vi "UHR-Fleezers Control (host) - 12.8.1.vi"() -> ()   [LabVIEW 2012] (continued)
                  frame Disabled {
                  }
                  frame Enabled {
                  }
                }
                n1750 = local read "Actual MCL Inc (V)"() -> (w2644:dbl)
                n1751 = local read "Scan steps (MCL)"() -> (w2649:u64)
                n1752 = Divide "Y Pix/step"(x=w2645, y=w2650) -> (x/y=w2657:dbl)
                n1753 = Divide "Y V/pix"(x=w2644, y=w2657) -> (x/y=w2656:dbl)
                n1754 = Divide "Y half step offset"(x=w2644, y=2.0) -> (x/y=w2658:dbl)
                n1755 = Divide "X pix/step"(x=w2646, y=w2649) -> (x/y=w2655:dbl)
                n1756 = Negate(x=w2658) -> (-x=w2659:dbl)
                n1757 = local read "Initial Y"() -> (w2665:dbl)
                n1758 = Multiply(x=w2647, y=w2656) -> (x*y=w2666:dbl)
                n1759 = Divide "X half step offset"(x=w2644, y=2.0) -> (x/y=w2652:dbl)
                n1760 = Divide "X V/pix"(x=w2644, y=w2655) -> (x/y=w2654:dbl)
                n1761 = Multiply(x=w2644, y=w2649) -> (x*y=w2661:dbl)
                n1762 = Compound Arithmetic op=ADD(w2659, w2666, w2665) -> (w2636:dbl)
                "Pointer Y (V)" <- w2636
                n1763 = Multiply(x=w2654, y=w2648) -> (x*y=w2663:dbl)
                n1764 = Negate(x=w2652) -> (-x=w2651:dbl)
                n1765 = local read "Initial X"() -> (w2664:dbl)
                n1766 = Negate(x=w2663) -> (-x=w2662:dbl)
                n1767 = Compound Arithmetic op=ADD(w2651, w2661, w2664, w2662) -> (w2637:dbl)
                "Pointer X (V)" <- w2637
                n1768 = case shown="True" "Set High F Confocal Spot (X-Y)" {
                  tunnel: w2637 -> [_ w2667]
                  tunnel: w2636 -> [_ w2668]
                  frame False {
                  }
                  frame True {
                    "Confocal Y 2 (V)" <- w2668
                    "Confocal X 2 (V)" <- w2667
                  }
                }
                n1769 = Or(x="Set X Only", y="Set Confocal Spot (X-Y)") -> (x .or. y?=w2640:bool)
                n1770 = Or(x="Set Confocal Spot (X-Y)", y="Set Y Only") -> (x .or. y?=w2639:bool)
                n1771 = case shown="True" w2640 {
                  tunnel: w2637 -> [_ w2669]
                  frame False {
                  }
                  frame True {
                    n1772 = property on="AO2" class="Slide (strict)"("Val(Sgnl)"=w2669) -> ()  [unwired: 2 in, 2 out]
                    "Confocal X 1 (V)" <- w2669
                  }
                }
                n1773 = case shown="True" w2639 {
                  tunnel: w2636 -> [_ w2670]
                  frame False {
                  }
                  frame True {
                    n1774 = property on="AO1" class="Slide (strict)"("Val(Sgnl)"=w2670) -> ()  [unwired: 2 in, 2 out]
                    "Confocal Y 1 (V)" <- w2670
                  }
                }
                n1775 = local write "Set High F Confocal Spot (X-Y)"(w2635) -> ()
                n1776 = local write "Set Confocal Spot (X-Y)"(w2635) -> ()
                n1777 = local write "Set X Only"(w2635) -> ()
                n1778 = local write "Set Y Only"(w2635) -> ()
              }
            }
          }
          frame 3 {
            n1779 = local read "BD 2 Frequency 1 (MHz)"() -> (w2672:dbl)
            n1780 = local read "BD 1 Frequency 1 (MHz)"() -> (w2673:dbl)
            n1781 = local write "Manipulating Trap"(TRUE ("Manipulating Trap")) -> ()
            n1782 = local write "Coords"(T9 {"Horizontal"=0, "Vertical"=0} ("Coords")) -> ()
            n1783 = while {
              tunnel: w2677 -> [w2682]
              tunnel: w2675 -> [w2681]
              tunnel: w2673 -> [w2680]
              tunnel: w2672 -> [w2679]
              tunnel: w2671 -> [w2678]
              stop <- w2683 stop-if-true
              n1784 = event shown="[0] \"Pane\": Mouse Move" {
                selector: _ -> [_ _]
                dyn-events: _ -> [_ _]
                timeout: _ -> [_ _]
                tunnel: ["Force Manip Abort" w2747] -> w2683
                tunnel: w2682 -> [w2690 _]
                tunnel: w2681 -> [w2688 _]
                tunnel: w2680 -> [w2687 _]
                tunnel: w2679 -> [w2686 _]
                tunnel: w2678 -> [w2684 _]
                event Mouse Move {
                  n1785 = event-data() -> ("Time"=w2691:u32, "Coords"=w2692:T9)  [unwired: 3 out]
                  n1786 = Less?(x=w2691, y=w2690) -> (x < y?=w2689:bool)
                  n1787 = case "Makes sure old motion events prior to mouse click aren't used" shown="False" w2689 {
                    tunnel: w2692 -> [w2734 _]
                    tunnel: w2688 -> [w2735 _]
                    tunnel: w2687 -> [w2709 _]
                    tunnel: w2686 -> [w2708 _]
                    tunnel: w2684 -> [w2693 _]
                    frame False {
                      n1788 = Subtract(x=w2734, y=w2735) -> (x-y=w2733:T9)
                      "Coords" <- w2733
                      n1789 = local read "Y RF Frequency Limits (MHz)"() -> (w2694:T18)
                      n1790 = To Double Precision Float(number=w2733) -> (double precision float=w2732:cluster{"Horizontal":dbl, "Vertical":dbl})
                      n1791 = Multiply(x=cluster{"Horizontal":dbl, "Vertical":dbl} {"Horizontal"=-1.0, "Vertical"=1.0}, y="Manipulation Scaling") -> (x*y=w2728:cluster{"Horizontal":dbl, "Vertical":dbl})
                      n1792 = local read "X RF Frequency Limits (MHz)"() -> (w2695:T18)
                      n1793 = Multiply(x=w2732, y=w2728) -> (x*y=w2730:cluster{"Horizontal":dbl, "Vertical":dbl})
                      n1794 = Unbundle By Name(w2730) -> ("Horizontal"=w2725:dbl, "Vertical"=w2729:dbl)
                      n1795 = Unbundle By Name(w2694) -> ("Maximum"=w2697:dbl, "Minimum"=w2696:dbl)
                      n1796 = Boolean To (0,1)(Boolean="Manip. X?") -> (0, 1=w2723:i16)
                      n1797 = Boolean To (0,1)(Boolean="Manip. Y?") -> (0, 1=w2720:i16)
                      n1798 = local read "BD 1 Frequency 2 (MHz)"() -> (w2711:dbl)
                      n1799 = Multiply(x=w2729, y=w2720) -> (x*y=w2722:dbl)
                      n1800 = Multiply(x=w2723, y=w2725) -> (x*y=w2726:dbl)
                      n1801 = local read "BD 2 Frequency 2 (MHz)"() -> (w2710:dbl)
                      n1802 = Unbundle By Name(w2695) -> ("Maximum"=w2699:dbl, "Minimum"=w2698:dbl)
                      n1803 = Add(x=w2708, y=w2722) -> (x+y=w2701:dbl)
                      n1804 = Add(x=w2709, y=w2726) -> (x+y=w2703:dbl)
                      n1805 = In Range and Coerce(upper limit=w2699, x=w2703, lower limit=w2698) -> (coerced(x)=w2702:dbl)  [unwired: 1 out]
                      n1806 = In Range and Coerce(upper limit=w2697, x=w2701, lower limit=w2696) -> (coerced(x)=w2700:dbl)  [unwired: 1 out]
                      n1807 = Subtract(x=w2702, y=w2711) -> (x-y=w2719:dbl)
                      n1808 = Subtract(x=w2700, y=w2710) -> (x-y=w2718:dbl)
                      n1809 = Square(x=w2719) -> (x^2=w2717:dbl)
                      n1810 = Square(x=w2718) -> (x^2=w2716:dbl)
                      n1811 = Add(x=w2717, y=w2716) -> (x+y=w2715:dbl)
                      n1812 = Square Root(x=w2715) -> (sqrt(x)=w2712:dbl)
                      n1813 = In Range and Coerce(upper limit="Limit Max (MHz)", x=w2712, lower limit="Limit Min (MHz)") -> (In Range?=w2705:bool)  [unwired: 1 out]
                      n1814 = Not(x="Limits Enable") -> (.not. x?=w2704:bool)
                      n1815 = Or(x=w2705, y=w2704) -> (x .or. y?=w2706:bool)
                      n1816 = case shown="True" w2706 {
                        tunnel: w2712 -> [_ w2737]
                        tunnel: w2702 -> [_ w2744]
                        tunnel: w2711 -> [_ w2743]
                        tunnel: w2700 -> [_ w2742]
                        tunnel: w2710 -> [_ w2741]
                        tunnel: w2695 -> [_ w2739]
                        tunnel: w2694 -> [_ w2738]
                        tunnel: w2693 -> [_ w2736]
                        frame False {
                        }
                        frame True {
                          n1817 = local read "BD 1 Frequency 3 (MHz)"() -> (w2745:dbl)
                          n1818 = local read "BD 2 Frequency 3 (MHz)"() -> (w2740:dbl)
                          n1819 = local write "Trap Delta (MHz)"(w2737) -> ()
                          n1820 = call "set RF board frequency - interlace.vi"("Board 2 Frequency Limits"=w2738, "Board 1 Frequency Limits"=w2739, "FPGA VI Reference In"=w2736, "Board 2 Frequency 3 (MHz)"=w2740, "Board 1 Frequency 3 (MHz)"=w2745, "Board 2 Frequency 2 (MHz)"=w2741, "Board 2 Frequency 1 (MHz)"=w2742, "Board 1 Frequency 2 (MHz)"=w2743, "Board 1 Frequency 1  (MHz)"=w2744) -> ()  [unwired: 1 in, 2 out]
                          n1821 = local write "BD 2 Frequency 1 (MHz)"(w2742) -> ()
                          n1822 = local write "BD 1 Frequency 1 (MHz)"(w2744) -> ()
                        }
                      }
                    }
                    frame True {
                    }
                  }
                }
                event Mouse Up {
                  n1823 = event-data() -> ("Button"=w2746:u16)  [unwired: 8 out]
                  n1824 = case shown="3" w2746 {
                    tunnel: [FALSE TRUE] -> w2747
                    frame 0, Default {
                    }
                    frame 3 {
                      n1825 = local read "Trap Delta (MHz)"() -> (w2749:dbl)
                      n1826 = property on="Initial delta (MHz)" class="DigNum (strict)"("Val(Sgnl)"=w2749) -> ()  [unwired: 2 in, 2 out]
                      n1827 = local write "Manipulating Trap"(FALSE ("Manipulating Trap")) -> ()
                    }
                  }
                }
              }
            }
          }
        }
      }
      event Mouse Move {
        n1828 = event-data() -> ()  [unwired: 6 out]
      }
    }
    n1829 = local read "Stop All"() -> (w2565:bool)
    n1830 = node-c288() -> ()  [unwired: 2 out]
  }
  n1831 = flat-sequence "Video" {
    tunnel: [w2762] -> w67
    tunnel: w67 -> [w2803]
    frame #0 {
      w2752 = FALSE ("File open?")
      n1832 = while {
        stop <- w2754 continue-if-true
        n1833 = call "Close Video Capture.vi"() -> ("error code OUT"=w2756:i32)
        n1834 = Equal?(x=w2756, y=0) -> (x = y?=w2754:bool)
      }
      n1835 = local write "New Video File"(w2752) -> ()
      n1836 = local write "File open?"(w2752) -> ()
      n1837 = local write "Save Video"(w2752) -> ()
      n1838 = local write "Stop All"(FALSE ("Stop All")) -> ()
    }
    frame #1 {
      n1839 = call "DMR_Init.vi"() -> ()  [unwired: 3 out]
    }
    frame #2 {
      w2757 = "DE245428202"  # MSU fleezers card #
      (unwired) "DE019116701"  # Illinois fleezers card #
      # "Setting the destination format to Mono8 makes sure that the image can be displayed in the intensity plot."
      n1840 = call "DMR_GetDevice.vi"("search string IN"=w2757) -> ("device handle OUT"=w2780:i32)  [unwired: 4 in, 2 out]
      n1841 = call "DMR_OpenDevice.vi"("device handle IN"=w2780) -> ("driver handle OUT"=w2763:i32)  [unwired: 4 out]
      n1842 = call "DMR_FindList.vi"("flags IN"=u32 0 ("flags"), "list name IN"="" ("String"), "list type IN"=T39."camera descriptions", "driver handle IN"=w2763) -> ("list handle OUT"=w2766:i32)  [unwired: 2 out]
      n1843 = call "DMR_FindList.vi"("flags IN"=u32 0 ("flags"), "list name IN"="Base", "list type IN"=T39."setting", "driver handle IN"=w2763) -> ("list handle OUT"=w2764:i32)  [unwired: 2 out]
      n1844 = call "OBJ_GetHandle.vi"("object name IN"="VideoStandard", "list handle IN"=w2766) -> ("object handle OUT"=w2760:i32)  [unwired: 3 out]
      n1845 = call "OBJ_GetHandle.vi"("object name IN"="PixelFormat", "list handle IN"=w2764) -> ("object handle OUT"=w2774:i32)  [unwired: 3 out]
      n1846 = call "OBJ_SetS.vi"("value index IN"=0, "value IN"="NTSC M", "object handle IN"=w2760) -> ()  [unwired: 2 out]
      n1847 = call "OBJ_SetS.vi"("value index IN"=0, "value IN"="Mono8" ("value"), "object handle IN"=w2774) -> ()  [unwired: 2 out]
      n1848 = call "OBJ_GetHandle.vi"("object name IN"="VideoChannel", "list handle IN"=w2764) -> ("object handle OUT"=w2770:i32)  [unwired: 3 out]
      n1849 = while {
        tunnel: [w2784] -> w2762
        tunnel: w2763 -> [w2781]
        stop <- w2782 continue-if-true
        n1850 = call "DMR_ImageRequestSingle.vi"("request control IN"=0, "driver handle IN"=w2781) -> ("error code OUT"=w2783:i32, "driver handle OUT"=w2784:i32)  [unwired: 2 out]
        n1851 = Equal To 0?(x=w2783) -> (x = 0?=w2782:bool)
      }
      n1852 = call "OBJ_SetI.vi"("value index IN"=0, "value IN"=3 ("Video channel"), "object handle IN"=w2770) -> ()  [unwired: 2 out]
    }
    frame #3 {
      w2791 = T23 0 items=["Grayscale (U8)", "Grayscale (I16)", "Grayscale (SGL)", "Complex (CSG)", "RGB (U32)", "HSL (U32)", "RGB (U64)"] ("Image Type")
      w2799 = T23 0 items=["Grayscale (U8)", "Grayscale (I16)", "Grayscale (SGL)", "Complex (CSG)", "RGB (U32)", "HSL (U32)", "RGB (U64)"] ("Image Type")
      n1853 = call "IMAQ AVI2 Get Codec Names"() -> ("Codec Names"=w2786:string[])  [unwired: 10 in, 1 out]
      "Installed Codec Names" <- w2786
      n1854 = for "Create Greyscale map" {
        N: 256 -> [_]
        tunnel: [w2805] -> w2788 mode=indexing
        workers-P: _ -> [_]
        i -> [w2808]
        n1855 = To Unsigned Byte Integer(number=w2808) -> (unsigned 8bit integer=w2804:u8)
        n1856 = Join Numbers(hi=w2804, lo=w2804) -> ((hi.lo)=w2807:u16)
        n1857 = Join Numbers(hi=w2804, lo=w2804) -> ((hi.lo)=w2806:u16)
        n1858 = Join Numbers(hi=w2807, lo=w2806) -> ((hi.lo)=w2805:u32)
      }
      n1859 = property on="Codec choice" class="CmbBox"("Strings[]"=w2786) -> ()  [unwired: 2 in, 2 out]
      n1860 = call "IMAQ Create"("Image Name"="Scaled video", "Image Type"=w2791) -> ("New Image"=w2790:T2)  [unwired: 2 in, 2 out]
      n1861 = call "IMAQ Create"("Image Name"="Main video", "Image Type"=w2799) -> ("New Image"=w2800:T2)  [unwired: 2 in, 2 out]
      n1862 = node-c288(0 ("Processor")) -> (w2798:T27)  [unwired: 3 out]
      n1863 = Initialize Array(u32 0 ("Window Number (0...15)"), 480 ("dimension size"), 640 ("dimension size")) -> (w2793:u32[][])
      n1864 = timed-loop {
        tunnel: w2803 -> [w2825]
        tunnel: [w2824] -> w2802
        tunnel: w2800 -> [w2823]
        timing: w2798 -> [_]
        timing-out: [_] -> w2797
        tunnel: w2793 -> [w2816]
        tunnel: w2790 -> [w2814]
        tunnel: w2788 -> [w2813]
        stop <- w2815 stop-if-true
        # "This block performs the \nactual image capture."
        n1865 = node-c288() -> (→"Finished Late? [i-1]":bool)  [unwired: 5 out]
        n1866 = local read "Stop All"() -> (w2815:bool)
        n1867 = feedback #1(T40 refnum ("AVI Refnum")) -> (w2821:T40)
        n1868 = case shown="True" "New Video File" {
          tunnel: [w2838 w2839] -> w2812
          tunnel: w2821 -> [w2838 w2840]
          frame False {
          }
          frame True {
            n1869 = flat-sequence {
              tunnel: w2840 -> [w2842]
              tunnel: [w2844] -> w2839
              frame #0 {
                n1870 = local read "File open?"() -> (w2841:bool)
                n1871 = case shown="True" w2841 {
                  tunnel: w2842 -> [_ w2843]
                  frame False {
                  }
                  frame True {
                    n1872 = call "IMAQ AVI2 Close"("AVI Refnum"=w2843) -> ()  [unwired: 10 in, 1 out]
                  }
                }
              }
              frame #1 {
                n1873 = local write "New Video File"(FALSE ("New Video File")) -> ()
                n1874 = call "Create new save file.vi"("Ext"=".avi" ("string"), "Index In"="Video Index") -> ("Path Out"=w2847:path, "Index Out"=w2849:dbl)  [unwired: 1 in]
                "Path Out" <- w2847
                n1875 = local write "Video Index"(w2849) -> ()
                n1876 = call "IMAQ AVI2 Create"("Codec"="Codec choice", "Frames Per Second"=u32 30, "AVI Path"=w2847) -> ("AVI Refnum"=w2844:T40)  [unwired: 7 in, 1 out]
                "File open?" <- TRUE ("Files open?")
              }
            }
          }
        }
        n1877 = feedback-in #1(w2812) -> ()
        n1878 = call "DMR_ImageRequestWaitFor.vi"("queue number IN"=0, "timeout(ms) IN"=500, "driver handle IN"=w2825) -> ("error code OUT"=w2829:i32, "request number OUT"=w2826:i32, "driver handle OUT"=w2827:i32)
        n1879 = Equal To 0?(x=w2829) -> (x = 0?=w2828:bool)
        n1880 = Reciprocal(x="Video Capture Rate (Hz)") -> (1/x=w2819:dbl)
        n1881 = Multiply(x=w2819, y=1000.0) -> (x*y=w2817:dbl)
        n1882 = case shown="True" w2828 {
          tunnel: w2827 -> [w2853 w2890]
          tunnel: w2826 -> [_ w2889]
          tunnel: [w2853 w2886] -> w2824
          tunnel: w2823 -> [_ w2872]
          tunnel: w2816 -> [_ w2875]
          tunnel: w2812 -> [_ w2855]
          tunnel: w2814 -> [_ w2869]
          tunnel: w2813 -> [_ w2868]
          frame False {
          }
          frame True {
            w2880 = u32 0 ("X-offset IN")
            n1883 = call "DMR_GetImageRequestBufferData.vi"("driver handle IN"=w2890, "request number IN"=w2889) -> ("width OUT"=w2879:i32, "height OUT"=w2878:i32, "driver handle OUT"=w2885:i32, "request number OUT"=w2884:i32, "bytes per pixel OUT"=w2881:i32)  [unwired: 13 out]
            n1884 = call "DMR_GetImageRequestBufferImageData.vi"("driver handle IN"=w2885, "request number IN"=w2884, "bytes per pixel IN"=w2881, "X-offset IN"=w2880, "Y-offset IN"=w2880, "height IN"=w2878, "width IN"=w2879) -> ("driver handle OUT"=w2883:u32, "request number OUT"=w2882:u32, "image OUT"=w2861:u32[][])  [unwired: 10 out]
            n1885 = Transpose 2D Array(2D array=w2861) -> (transposed array=w2867:u32[][])
            n1886 = Select(t=w2867, s="Flip Y (or X)", f=w2861) -> (s? t:f=w2866:u32[][])
            n1887 = call "DMR_ImageRequestUnlock.vi"("request number IN"=w2882, "driver handle IN"=w2883) -> ("driver handle OUT"=w2888:i32)  [unwired: 1 in, 2 out]
            n1888 = for {
              tunnel: w2866 -> [w2925] mode=indexing
              tunnel: [w2924] -> w2864 mode=indexing
              n1889 = Reverse 1D Array(array=w2925) -> (reversed array=w2924:u32[])
            }
            n1890 = call "DMR_ImageRequestSingle.vi"("request control IN"=0, "driver handle IN"=w2888) -> ("driver handle OUT"=w2886:i32)  [unwired: 3 out]
            n1891 = Transpose 2D Array(2D array=w2864) -> (transposed array=w2865:u32[][])
            n1892 = Select(t=w2865, s="Flip Y (or X)", f=w2864) -> (s? t:f=w2862:u32[][])
            n1893 = Select(t=w2862, s="Flip Image", f=w2861) -> (s? t:f=w2859:u32[][])
            n1894 = case shown="True" "Averaging" {
              tunnel: w2859 -> [w2936 w2941]
              tunnel: [w2936 w2940] -> w2873
              tunnel: w2875 -> [_ w2938]
              frame False {
              }
              frame True {
                (unwired) 1
                w2946 = 1
                n1895 = feedback #2(w2938) -> (w2937:u32[][])
                n1896 = Add(x=w2941, y=w2937) -> (x+y=w2942:u32[][])
                n1897 = Select(t=w2938, s="Reset Averaging", f=w2942) -> (s? t:f=w2944:u32[][])
                n1898 = feedback-in #2(w2944) -> ()
                n1899 = feedback #3(w2946) -> (w2939:i32)
                n1900 = Divide(x=w2942, y=w2939) -> (x/y=w2943:dbl[][])
                n1901 = Increment(x=w2939) -> (x+1=w2947:i32)
                n1902 = To Unsigned Long Integer(number=w2943) -> (unsigned 32bit integer=w2940:u32[][])
                n1903 = Select(t=w2946, s="Reset Averaging", f=w2947) -> (s? t:f=w2945:i32)
                n1904 = feedback-in #3(w2945) -> ()
              }
            }
            n1905 = case shown="True" "Zoom video window" {
              tunnel: w2873 -> [_ w2904]
              tunnel: w2869 -> [_ w2903]
              frame False {
              }
              frame True {
                n1906 = To Double Precision Float(number=w2904) -> (double precision float=w2901:dbl[][])
                n1907 = In Range and Coerce(upper limit="Intensity Upper", x=w2901, lower limit="Intensity Lower") -> (coerced(x)=w2900:dbl[][])  [unwired: 1 out]
                n1908 = Subtract(x="Intensity Upper", y="Intensity Lower") -> (x-y=w2897:dbl)
                n1909 = Subtract(x=w2900, y="Intensity Lower") -> (x-y=w2898:dbl[][])
                n1910 = Divide(x=w2898, y=w2897) -> (x/y=w2899:dbl[][])
                n1911 = Multiply(x=255.0, y=w2899) -> (x*y=w2895:dbl[][])
                n1912 = To Unsigned Byte Integer(number=w2895) -> (unsigned 8bit integer=w2902:u8[][])
                n1913 = call "IMAQ ArrayToImage"("Image Pixels (U8)"=w2902, "Image"=w2903) -> ("Image Out"=w2891:T2)  [unwired: 4 in, 5 out]
                n1914 = First Call?() -> (First Call?: T/F=w2892:bool)
                n1915 = case shown="True" w2892 {
                  tunnel: w2891 -> [w2905 w2916]
                  frame False {
                    n1916 = flat-sequence {
                      tunnel: w2905 -> [w2911]
                      frame #0 {
                        w2908 = FALSE ("Get/Set Status? (Set)")
                        w2907 = 0 ("Window Number (0...15)")
                        n1917 = call "IMAQ WindSize"("Get/Set Status? (Set)"=w2908, "Window Number"=w2907) -> ("Width & Height out"=→"Window Size":cluster{"Width":i32, "Height":i32})  [unwired: 4 in, 2 out]
                        n1918 = call "IMAQ WindMove"("Window Number (0...15)"=w2907, "Get/Set Status? (Set)"=w2908) -> ("Coordinates (screen)"=→"Window Position":cluster{"X Position":i32, "Y Position":i32})  [unwired: 3 in, 1 out]
                        n1919 = call "IMAQ WindDraw"("Resize to Image Size? (Y)"=FALSE, "Window Number (0...15)"=w2907, "Image"=w2911) -> ()  [unwired: 7 in, 2 out]
                      }
                      frame #1 {
                        n1920 = call "IMAQ WindZoom 2"("Center Point"="Center Point", "Zoom to Fit? (False)"=FALSE, "Zoom Factor"="Zoom Factor") -> ()  [unwired: 5 in, 4 out]
                      }
                    }
                  }
                  frame True {
                    n1921 = flat-sequence {
                      tunnel: w2916 -> [w2919]
                      tunnel: [w2917] -> w2915
                      tunnel: w2915 -> [w2921]
                      frame #0 {
                        w2918 = TRUE ("Resize to Image Size? (Y)")
                        w2917 = 0 ("Window Number (0...15)")
                        n1922 = call "IMAQ WindNonTearing"("Window Number"=w2917, "NonTearing? (True)"=w2918) -> ()  [unwired: 8 in, 2 out]
                        n1923 = call "IMAQ WindDraw"("Resize to Image Size? (Y)"=w2918, "Window Number (0...15)"=w2917, "Image"=w2919) -> ()  [unwired: 7 in, 2 out]
                      }
                      frame #1 {
                        n1924 = call "IMAQ WindSize"("Scrollbars? (N)"=FALSE, "Width & Height"="Initial Window Size", "Window Number"=w2921) -> ()  [unwired: 3 in, 3 out]
                        n1925 = call "IMAQ WindMove"("Window Number (0...15)"=w2921, "Coordinates (screen)"="Initial Window Position") -> ()  [unwired: 3 in, 2 out]
                      }
                    }
                  }
                }
              }
            }
            n1926 = To Unsigned Byte Integer(number=w2873) -> (unsigned 8bit integer=w2871:u8[][])
            n1927 = call "IMAQ ArrayToImage"("Image Pixels (U8)"=w2871, "Image"=w2872) -> ("Image Out"=w2870:T2)  [unwired: 4 in, 5 out]
            "Primary Video Display" <- w2870
            n1928 = Not(x="Close Video File") -> (.not. x?=w2857:bool)
            n1929 = And(x="Save Video", y=w2857) -> (x .and. y?=w2854:bool)
            n1930 = case shown="True" "Save Image" {
              tunnel: w2871 -> [_ w2950]
              tunnel: w2868 -> [_ w2949]
              frame False {
              }
              frame True {
                n1931 = call <vilib>:"Flatten Pixmap.vi"("colors"=w2949, "8-bit pixmap"=w2950) -> ("image data"=w2956:T41)  [unwired: 4 in, 5 out]
                n1932 = call "Create new save file.vi"("Insert"="video_frame_" ("string"), "Ext"=".bmp" ("string"), "Index In"="Image Index") -> ("Path Out"=w2952:path, "Index Out"=w2957:dbl)
                n1933 = Increment(x=w2957) -> (x+1=w2951:dbl)
                n1934 = local write "Image Index"(w2951) -> ()
                n1935 = call <vilib>:"Write BMP File.vi"("image data"=w2956, "path to BMP file"=w2952) -> ()  [unwired: 1 in, 9 out]
              }
            }
            n1936 = case shown="True" w2854 {
              tunnel: w2855 -> [w2927 w2932]
              tunnel: w2870 -> [_ w2931]
              tunnel: "Close Video File" -> [w2926 _]
              frame False {
                n1937 = case shown="True" w2926 {
                  tunnel: w2927 -> [_ w2928]
                  frame False {
                  }
                  frame True {
                    w2929 = FALSE ("Save Video")
                    n1938 = call "IMAQ AVI2 Close"("AVI Refnum"=w2928) -> ()  [unwired: 10 in, 1 out]
                    n1939 = local write "File open?"(w2929) -> ()
                    n1940 = local write "Save Video"(w2929) -> ()
                  }
                }
              }
              frame True {
                n1941 = local read "File open?"() -> (w2930:bool)
                n1942 = case shown="True" w2930 {
                  tunnel: w2932 -> [_ w2935]
                  tunnel: w2931 -> [_ w2934]
                  frame False {
                    n1943 = local write "New Video File"(TRUE ("New Video File")) -> ()
                  }
                  frame True {
                    n1944 = call "IMAQ AVI2 Write Frame"("Image"=w2934, "AVI Refnum"=w2935) -> ()  [unwired: 7 in, 3 out]
                  }
                }
              }
            }
          }
        }
        n1945 = node-c288(w2817, "Deadline (ms)") -> ()  [unwired: 1 out]
      }
      n1946 = node-c288(w2797) -> ()  [unwired: 1 out]
      n1947 = call "DMR_CloseDevice.vi"("driver handle IN"=w2802) -> ()  [unwired: 1 in, 4 out]
    }
    frame #4 {
      n1948 = call "DMR_Close.vi"() -> ()  [unwired: 1 out]
    }
  }
  n1949 = node-c288(3 ("Processor")) -> (w76:T27)  [unwired: 3 out]
  n1950 = timed-loop "Oscillate Trap/AOM (fishing, conjugate plane alignment)" {
    tunnel: [w2963] -> w81
    timing: w76 -> [_]
    timing-out: [_] -> w75
    tunnel: w17 -> [w2962]
    stop <- w2963 stop-if-true
    n1951 = node-c288() -> ()  [unwired: 2 out]
    n1952 = event shown="[0] \"Oscillate Set 1\", \"Fish for Tether\": Value Change" {
      selector: _ -> [_ _ _]
      dyn-events: _ -> [_ _ _]
      timeout: _ -> [_ _ _]
      tunnel: [FALSE ("Stop All") _ w3570] -> w2963
      tunnel: w2962 -> [w2966 _ _]
      event "Oscillate Set 1", "Fish for Tether": Value Change {
        n1953 = event-data() -> ()  [unwired: 6 out]
        n1954 = local read "Oscillate Set 1"() -> (w2970:bool)
        n1955 = Or(x=w2970, y="Fish for Tether") -> (x .or. y?=w2968:bool)
        n1956 = case shown="True" w2968 {
          tunnel: "Fish for Tether" -> [_ w2973]
          tunnel: w2966 -> [_ w2971]
          frame False {
          }
          frame True {
            n1957 = case shown="True" w2973 {
              selector: w2973 -> [w2976 w2982]
              tunnel: [w2976 w2982] -> w2972
              frame False {
              }
              frame True {
                n1958 = local write "Scan axis 2"(TRUE) -> ()
                n1959 = local write "Tether"(FALSE ("Tether")) -> ()
                n1960 = local read "Flow ON during cal?"() -> (w2977:bool)
                n1961 = property on="Trap Delta (MHz)" class="DigNum (strict)"("Val(Sgnl)"="Furthest Delta (MHz)") -> ()  [unwired: 2 in, 2 out]
                n1962 = Or(x="Flow ON during \nfishing?", y=w2977) -> (x .or. y?=w2978:bool)
                n1963 = Wait (ms)(milliseconds to wait=u32 500) -> ()  [unwired: 1 out]
                n1964 = property on="Sample Channel\nFlow" class="Bool (strict)"("Val(Sgnl)"=w2978) -> ()  [unwired: 2 in, 2 out]
              }
            }
            n1965 = node-c288() -> (w2975:T27)  [unwired: 1 in, 3 out]
            n1966 = timed-loop "Oscillate AOD" {
              timing: w2975 -> [_]
              timing-out: [_] -> w2974
              tunnel: w2972 -> [w2986]
              tunnel: w2971 -> [w2985]
              i -> [w2994]
              stop <- w2992 stop-if-true
              n1967 = node-c288() -> (w2993:i64)  [unwired: 1 out]
              n1968 = flat-sequence {
                tunnel: w2994 -> [w3021]
                tunnel: w2993 -> [w3020]
                tunnel: w2986 -> [w3004]
                tunnel: [w3004] -> w2991
                tunnel: [w3003] -> w2990
                tunnel: [w3002] -> w2989
                tunnel: [w2999] -> w2987
                tunnel: w2985 -> [w2995]
                tunnel: w2991 -> [w3068]
                tunnel: w2990 -> [w3066]
                tunnel: w2989 -> [w3065]
                tunnel: [w3064] -> w2988
                tunnel: w2987 -> [w3063]
                tunnel: [w3140] -> w2992
                tunnel: w2988 -> [w3139]
                frame #0 {
                  # "w (rad/s)"
                  # "t (s)"
                  n1969 = Divide(x=w3020, y=i64 1000) -> (x/y=w2996:dbl)
                  n1970 = local read "BD 1 Frequency 2 (MHz)"() -> (w2998:dbl)
                  n1971 = Multiply(x="Osc. freq. (Hz)", y=6.283185307179586) -> (x*y=w3018:dbl)
                  n1972 = Multiply(x=w2996, y=w3021) -> (x*y=w3017:dbl)
                  n1973 = Multiply(x=w3018, y=w3017) -> (x*y=w3001:dbl)
                  n1974 = local read "BD 1 Frequency 1 (MHz)"() -> (w3006:dbl)
                  n1975 = case shown="True" w3004 {
                    tunnel: w3001 -> [w3027 w3046]
                    tunnel: w3006 -> [_ w3054]
                    tunnel: w2998 -> [_ w3055]
                    tunnel: [w3024 w3050] -> w2997
                    tunnel: [FALSE w3028] -> w3002
                    tunnel: [0.0 w3042] -> w2999
                    frame False {
                      n1976 = Sine(x=w3027) -> (sin(x)=w3025:dbl)
                      n1977 = Multiply(x=w3025, y="Osc. amp. (MHz)") -> (x*y=w3024:dbl)
                    }
                    frame True {
                      # "trap position goes from 0 to 1 (0 is when it is furthest away, 1 is when closest)\nso we want to test for tether only when farther away, or x < 1"
                      # "quit if taking too long"
                      # "oscillate the trap"
                      # "Test for tether"
                      n1978 = local read "Vec Mean of T1 T2"() -> (w3031:dbl[])
                      "Trigger Signal" <- w3031
                      n1979 = Cosine(x=w3046) -> (cos(x)=w3058:dbl)
                      n1980 = Subtract(x=w3055, y=w3054) -> (x-y=w3053:dbl)
                      n1981 = Decrement(x=w3058) -> (x-1=w3057:dbl)
                      n1982 = Subtract(x=w3053, y="Closest Delta (MHz)") -> (x-y=w3051:dbl)
                      n1983 = Divide(x=w3057, y=-2.0) -> (x/y=w3041:dbl)
                      n1984 = Greater?(x=w3031, y="Stop F (pN)") -> (0:w3048:bool[])
                      n1985 = Multiply(x=w3041, y=w3051) -> (x*y=w3050:dbl)
                      n1986 = Less?(x=w3041, y="Fish mask thresh") -> (x < y?=w3040:bool)
                      n1987 = Boolean To (0,1)(Boolean=w3040) -> (0, 1=w3038:i16)
                      n1988 = Multiply(x=w3038, y=w3031) -> (x*y=w3037:dbl[])
                      n1989 = Divide(x=w3046, y=6.283185307179586) -> (x/y=w3045:dbl)
                      n1990 = Round Toward +Infinity(x=w3045) -> (ceil(x): smallest int >= x=w3042:dbl)
                      "Attempts" <- w3042
                      n1991 = Greater?(x=w3037, y="Stop F (pN) (mask)") -> (0:w3035:bool[])
                      n1992 = Or Array Elements(Boolean array=w3048) -> (logical OR=w3033:bool)
                      n1993 = Or Array Elements(Boolean array=w3035) -> (logical OR=w3032:bool)
                      n1994 = Greater?(x=w3042, y="Attempt Limit") -> (0:w3044:bool)
                      n1995 = case shown="True" w3044 {
                        frame False {
                        }
                        frame True {
                          n1996 = local write "Fish for Tether"(FALSE ("Fish for Tether")) -> ()
                          n1997 = call <vilib>:"Beep.vi"() -> ()  [unwired: 3 in, 9 out]
                          n1998 = local read "Messages"() -> (w3060:string)
                          n1999 = call "Update messages.vi"("Message to add"="Tether fishing timeout." ("Messages"), "Old message string"=w3060) -> ("New message string"=→"Messages":string)
                        }
                      }
                      n2000 = Select(t=w3033, s="Normal (on) or masked test (off)", f=w3032) -> (s? t:f=w3030:bool)
                      n2001 = And(x="Stop Fishing When Tether", y=w3030) -> (x .and. y?=w3028:bool)
                    }
                  }
                  n2002 = local read "BD 2 Frequency 1 (MHz)"() -> (w3005:dbl)
                  n2003 = Select(t=w3006, s="Scan axis 2", f=w3005) -> (s? t:f=w3009:dbl)
                  n2004 = Add(x=w2997, y=w3009) -> (x+y=w3003:dbl)
                  n2005 = Select(t=w3003, s="Scan axis 2", f=w3006) -> (s? t:f=w3012:dbl)
                  n2006 = Select(t=w3005, s="Scan axis 2", f=w3003) -> (s? t:f=w3011:dbl)
                  n2007 = local read "BD 2 Frequency 2 (MHz)"() -> (w3014:dbl)
                  n2008 = local read "BD 2 Frequency 3 (MHz)"() -> (w3013:dbl)
                  n2009 = local read "Y RF Frequency Limits (MHz)"() -> (w3007:T18)
                  n2010 = local read "X RF Frequency Limits (MHz)"() -> (w3008:T18)
                  n2011 = local read "BD 1 Frequency 3 (MHz)"() -> (w3015:dbl)
                  n2012 = call "set RF board frequency - interlace.vi"("Board 2 Frequency Limits"=w3007, "Board 1 Frequency Limits"=w3008, "FPGA VI Reference In"=w2995, "Board 2 Frequency 3 (MHz)"=w3013, "Board 1 Frequency 3 (MHz)"=w3015, "Board 2 Frequency 2 (MHz)"=w3014, "Board 2 Frequency 1 (MHz)"=w3011, "Board 1 Frequency 2 (MHz)"=w2998, "Board 1 Frequency 1  (MHz)"=w3012) -> ()  [unwired: 1 in, 2 out]
                }
                frame #1 {
                  n2013 = And(x=w3068, y=w3065) -> (x .and. y?=w3067:bool)
                  n2014 = case "Only if were fishing and now formed tether" shown="True" w3067 {
                    tunnel: w3066 -> [w3070 w3085]
                    tunnel: [w3069 w3084] -> w3064
                    tunnel: w3063 -> [_ w3080]
                    frame False {
                      n2015 = local read "Fish for Tether"() -> (w3069:bool)
                      n2016 = case shown="False" w3069 {
                        tunnel: w3070 -> [w3071 _]
                        frame False {
                          n2017 = property on="BD 1 Frequency 1 (MHz)" class="DigNum (strict)"("Val(Sgnl)"=w3071) -> ()  [unwired: 2 in, 2 out]
                        }
                        frame True {
                        }
                      }
                    }
                    frame True {
                      w3084 = FALSE ("Fish for Tether")
                      n2018 = call <vilib>:"Beep.vi"() -> ()  [unwired: 3 in, 9 out]
                      n2019 = Number To Decimal String(number=w3080, width (-)=i16 1) -> (decimal integer string=w3078:string)
                      n2020 = Concatenate Strings("Formed tether in ", w3078, " attempt(s)." ("string")) -> (w3075:string)
                      n2021 = local read "Messages"() -> (w3082:string)
                      n2022 = local write "Fish for Tether"(w3084) -> ()
                      n2023 = call "Update messages.vi"("Message to add"=w3075, "Old message string"=w3082) -> ("New message string"=w3081:string)
                      n2024 = local write "Messages"(w3081) -> ()
                      n2025 = Get Date/Time In Seconds() -> (seconds since 1Jan1904=→"Time tether formed":timestamp)
                      n2026 = local read "Flow ON during cal?"() -> (w3072:bool)
                      n2027 = property on="Sample Channel\nFlow" class="Bool (strict)"("Val(Sgnl)"=w3072) -> (error out=w3073:errorcluster)  [unwired: 2 in, 1 out]
                      n2028 = case shown="\"2\", \"3\", \"4\", \"5\", \"6\"" "Then..." {
                        selector: "Then..." -> [_ w3088]
                        tunnel: w3085 -> [w3087 _]
                        tunnel: w3073 -> [_ _]
                        frame "1", Default {
                          n2029 = property on="BD 1 Frequency 1 (MHz)" class="DigNum (strict)"("Val(Sgnl)"=w3087) -> ()  [unwired: 2 in, 2 out]
                        }
                        frame "2", "3", "4", "5", "6" {
                          n2030 = flat-sequence {
                            tunnel: w3088 -> [w3090]
                            frame #0 {
                              n2031 = property on="Trap Delta (MHz)" class="DigNum (strict)"("Val(Sgnl)"="Move to Delta 1 (MHz)") -> ()  [unwired: 2 in, 2 out]
                            }
                            frame #1 {
                              n2032 = case shown="\"5\", \"6\"" w3090 {
                                selector: w3090 -> [w3093 w3103 _]
                                frame "3", "4" {
                                n2033 = flat-sequence {
                                tunnel: w3093 -> [w3094]
                                tunnel: [w3094] -> w3091
                                tunnel: [w3096] -> w3092
                                tunnel: w3091 -> [w3096]
                                tunnel: w3092 -> [w3100]
                                frame #0 {
                                n2034 = property on="Green Laser ON" class="Bool (strict)"("Val(Sgnl)"=TRUE ("Value (Signaling)")) -> ()  [unwired: 2 in, 2 out]
                                }
                                frame #1 {
                                n2035 = Multiply(x="Wait Before Save (s)", y=u32 1000 ("x")) -> (x*y=w3098:u32)
                                n2036 = Wait (ms)(milliseconds to wait=w3098) -> ()  [unwired: 1 out]
                                }
                                frame #2 {
                                n2037 = property on="Start Saving" class="Bool (strict)"("Value"=TRUE ("Start Saving")) -> ()  [unwired: 2 in, 2 out]
                                n2038 = case shown="\"4\"" w3100 {
                                frame Default {
                                }
                                frame "4" {
                                n2039 = property on="Fl. Triggered..." class="Bool (strict)"("Val(Sgnl)"=TRUE ("Value (Signaling)")) -> ()  [unwired: 2 in, 2 out]
                                }
                                }
                                }
                                }
                                }
                                frame "5", "6" {
                                n2040 = stacked-sequence {
                                tunnel: w3103 -> [_ _ _ _ _ _ w3115]
                                frame #0 {
                                n2041 = Replace Array Subset(array=u32[] [0] ("Index Values"), new element="Raster Set Upon Tether", index=0) -> (w3104:u32[])
                                n2042 = property on="Saved AOD Raster Scan Parameter Sets" class="Arr (strict)"("Index Values"=w3104) -> ()  [unwired: 2 in, 2 out]
                                }
                                frame #1 {
                                n2043 = Wait (ms)(milliseconds to wait=u32 500) -> ()  [unwired: 1 out]
                                }
                                frame #2 {
                                n2044 = property on="Load parameters" class="Bool (strict)"("Val(Sgnl)"=TRUE ("Value (Signaling)")) -> ()  [unwired: 2 in, 2 out]
                                n2045 = case shown="True" "Green ON During Raster" {
                                frame False {
                                }
                                frame True {
                                n2046 = property on="Green Laser ON" class="Bool (strict)"("Val(Sgnl)"=TRUE ("Value (Signaling)")) -> ()  [unwired: 2 in, 2 out]
                                }
                                }
                                }
                                frame #3 {
                                n2047 = Wait (ms)(milliseconds to wait=u32 500) -> ()  [unwired: 1 out]
                                }
                                frame #4 {
                                n2048 = property on="Trap Raster Scan" class="Bool (strict)"("Val(Sgnl)"=TRUE ("Value (Signaling)")) -> ()  [unwired: 2 in, 2 out]
                                }
                                frame #5 {
                                n2049 = Wait (ms)(milliseconds to wait=u32 2000) -> ()  [unwired: 1 out]
                                }
                                frame #6 {
                                n2050 = flat-sequence {
                                tunnel: w3115 -> [w3122]
                                frame #0 {
                                n2051 = while {
                                stop <- w3118 stop-if-true
                                n2052 = local read "Raster Scanning..."() -> (w3117:bool)
                                n2053 = local read "Saving..."() -> (w3120:bool)
                                n2054 = Wait (ms)(milliseconds to wait=u32 100) -> ()  [unwired: 1 out]
                                n2055 = Not(x=w3120) -> (.not. x?=w3119:bool)
                                n2056 = Not(x=w3117) -> (.not. x?=w3116:bool)
                                n2057 = And(x=w3119, y=w3116) -> (x .and. y?=w3118:bool)
                                }
                                }
                                frame #1 {
                                n2058 = local read "Tether"() -> (w3123:bool)
                                n2059 = case shown="True" w3123 {
                                tunnel: w3122 -> [_ w3125]
                                frame False {
                                n2060 = property on="Fish for Tether" class="Bool (strict)"("Val(Sgnl)"="Fish again after \nraster break?") -> ()  [unwired: 2 in, 2 out]
                                }
                                frame True {
                                n2061 = stacked-sequence {
                                tunnel: w3125 -> [_ w3129 _ _]
                                frame #0 {
                                n2062 = property on="Trap Delta (MHz)" class="DigNum (strict)"("Val(Sgnl)"="Move to Delta 2 (MHz)") -> ()  [unwired: 2 in, 2 out]
                                n2063 = case shown="True" "Flow ON after\ntether testing?" {
                                frame False {
                                }
                                frame True {
                                n2064 = property on="Sample Channel\nFlow" class="Bool (strict)"("Val(Sgnl)"=TRUE ("Value (Signaling)")) -> ()  [unwired: 2 in, 2 out]
                                }
                                }
                                }
                                frame #1 {
                                n2065 = flat-sequence {
                                tunnel: w3129 -> [w3131]
                                frame #0 {
                                n2066 = Wait (ms)(milliseconds to wait=u32 500) -> ()  [unwired: 1 out]
                                }
                                frame #1 {
                                n2067 = case shown="\"6\"" w3131 {
                                frame Default {
                                }
                                frame "6" {
                                n2068 = property on="Green Laser ON" class="Bool (strict)"("Val(Sgnl)"=TRUE ("Green Laser ON/Interlacing")) -> ()  [unwired: 2 in, 2 out]
                                }
                                }
                                }
                                frame #2 {
                                n2069 = Wait (ms)(milliseconds to wait=u32 500) -> ()  [unwired: 1 out]
                                }
                                frame #3 {
                                n2070 = local write "Start Saving"("Save at end (5, 6)") -> ()
                                }
                                }
                                }
                                frame #2 {
                                n2071 = local read "Bead Sep. Int. Time (s)"() -> (w3137:dbl)
                                n2072 = Multiply(x=w3137, y=1000.0) -> (x*y=w3136:dbl)
                                n2073 = Wait (ms)(milliseconds to wait=w3136) -> ()  [unwired: 1 out]
                                }
                                frame #3 {
                                n2074 = property on="Remove Offset" class="Bool (strict)"("Val(Sgnl)"=TRUE ("Value (Signaling)")) -> ()  [unwired: 2 in, 2 out]
                                }
                                }
                                }
                                }
                                }
                                }
                                }
                                }
                                }
                                frame "2", Default {
                                }
                              }
                            }
                          }
                        }
                      }
                      "Tether" <- "Tether Alarm?"
                    }
                  }
                }
                frame #2 {
                  n2075 = local read "Oscillate Set 1"() -> (w3144:bool)
                  n2076 = local read "Stop All"() -> (w3142:bool)
                  n2077 = Or(x=w3144, y=w3139) -> (x .or. y?=w3141:bool)
                  n2078 = Not(x=w3141) -> (.not. x?=w3143:bool)
                  n2079 = Compound Arithmetic op=OR(w3142, w3143) -> (w3140:bool)
                }
              }
              n2080 = node-c288() -> ()  [unwired: 2 out]
            }
            n2081 = node-c288(w2974) -> ()  [unwired: 1 out]
          }
        }
      }
      event "Fl. Triggered...": Value Change {
        n2082 = event-data() -> ()  [unwired: 7 out]
        n2083 = case shown="True" "Fl. Triggered..." {
          frame False {
          }
          frame True {
            n2084 = node-c288() -> (w3155:T27)  [unwired: 4 out]
            n2085 = timed-loop {
              timing: w3155 -> [_]
              timing-out: [_] -> w3154
              tunnel: "Action" -> [w3163]
              shift-right: [w3160] -> _
              shift-left: u8 255 -> [w3162]
              shift-right: [w3157] -> _
              shift-left: 255 -> [w3159]
              stop <- w3156 stop-if-true
              # "Reset confocal spot"
              n2086 = node-c288() -> ()  [unwired: 2 out]
              n2087 = flat-sequence {
                tunnel: w3163 -> [w3183]
                tunnel: w3162 -> [w3182]
                tunnel: [w3181] -> w3161
                tunnel: w3159 -> [w3168]
                tunnel: [w3167] -> w3158
                tunnel: [w3562] -> w3156
                tunnel: w3161 -> [w3561]
                tunnel: [w3561] -> w3160
                tunnel: [w3560] -> w3157
                tunnel: w3158 -> [w3560]
                frame #0 {
                  n2088 = local read "Delta Fl. 2"() -> (w3180:dbl)
                  n2089 = local read "Delta Fl. 1"() -> (w3175:dbl)
                  n2090 = Multiply(x="Fl. Delta Thresh. (kHz)", y=1000.0) -> (x*y=w3170:dbl)
                  n2091 = Select(t=w3175, s="APD to Watch", f=w3180) -> (s? t:f=w3171:dbl)
                  n2092 = Greater?(x=w3171, y=w3170) -> (0:w3176:bool)
                  n2093 = Or(x="Force Yank", y=w3176) -> (x .or. y?=w3174:bool)
                  n2094 = And(x=w3174, y="Yank when?") -> (x .and. y?=w3172:bool)
                  n2095 = case shown="False" w3172 {
                    tunnel: w3183 -> [w3186 w3387]
                    tunnel: w3182 -> [w3188 w3383]
                    tunnel: [w3188 w3381] -> w3181
                    tunnel: w3171 -> [w3194 _]
                    tunnel: w3170 -> [w3193 _]
                    tunnel: "Force Yank" -> [w3191 _]
                    tunnel: w3168 -> [w3190 w3380]
                    tunnel: [w3189 w3380] -> w3167
                    frame False {
                      n2096 = Negate(x=w3193) -> (-x=w3185:dbl)
                      n2097 = local write "Fl. High"(TRUE ("Fl. High")) -> ()
                      n2098 = Less?(x=w3194, y=w3185) -> (x < y?=w3192:bool)
                      n2099 = Or(x=w3191, y=w3192) -> (x .or. y?=w3187:bool)
                      n2100 = case shown="True" w3187 {
                        tunnel: w3190 -> [w3195 w3205]
                        tunnel: [w3195 w3204] -> w3189
                        tunnel: w3186 -> [_ w3203]
                        frame False {
                        }
                        frame True {
                          n2101 = flat-sequence {
                            tunnel: w3205 -> [w3211]
                            tunnel: w3203 -> [w3208]
                            tunnel: [w3210] -> w3202
                            tunnel: [w3209] -> w3201
                            tunnel: [w3208] -> w3200
                            tunnel: w3199 -> [w3207]
                            tunnel: [w3207] -> w3198
                            tunnel: w3197 -> [w3206]
                            tunnel: [w3206] -> w3196
                            tunnel: [w3282] -> w3204
                            tunnel: w3202 -> [w3282]
                            tunnel: w3201 -> [w3281]
                            tunnel: w3200 -> [w3280]
                            tunnel: w3198 -> [w3279]
                            tunnel: w3196 -> [w3278]
                            frame #0 {
                              n2102 = call <vilib>:"Beep.vi"() -> ()  [unwired: 12 in]
                              n2103 = local write "Waiting"(FALSE ("Waiting")) -> ()
                              n2104 = Increment(x=w3211) -> (x+1=w3210:i32)
                              n2105 = case shown="\"Image\"" w3208 {
                                tunnel: w3210 -> [_ w3216 _]
                                frame "Alarm", Default {
                                }
                                frame "Yank" {
                                n2106 = flat-sequence {
                                tunnel: w3216 -> [w3219]
                                tunnel: [w3218] -> w3215
                                tunnel: [w3217] -> w3214
                                tunnel: w3215 -> [w3229]
                                tunnel: w3214 -> [w3230]
                                frame #0 {
                                n2107 = local read "Yank Delay (s)"() -> (w3222:dbl)
                                n2108 = local read "N Array El"() -> (w3217:u8)
                                n2109 = Quotient & Remainder(x=w3219, y=w3217) -> (x-y*floor(x/y)=w3218:i32)  [unwired: 1 out]
                                n2110 = Multiply(x=w3222, y=1000.0) -> (x*y=w3220:dbl)
                                n2111 = Wait (ms)(milliseconds to wait=w3220) -> ()  [unwired: 1 out]
                                }
                                frame #1 {
                                n2112 = local read "Yank to which?"() -> (w3224:bool)
                                n2113 = local read "Random Choice"() -> (w3234:bool)
                                n2114 = local read "Yank to Trap Delta (MHz)"() -> (w3227:dbl[])
                                n2115 = local read "Yank to SP"() -> (w3228:dbl[])
                                n2116 = Random Number (0-1)() -> (number: 0 to 1=w3233:dbl)
                                n2117 = Multiply(x=w3230, y=w3233) -> (x*y=w3232:dbl)
                                n2118 = Round Toward -Infinity(1:w3232) -> (0:w3231:dbl)
                                n2119 = Select(t=w3231, s=w3234, f=w3229) -> (s? t:f=w3225:dbl)
                                n2120 = Select(t=w3227, s=w3224, f=w3228) -> (s? t:f=w3226:dbl[])
                                n2121 = Index Array(array=w3226, index=w3225) -> (element=w3223:dbl)
                                n2122 = case shown="True" w3224 {
                                tunnel: w3223 -> [w3235 w3262]
                                frame False {
                                n2123 = flat-sequence {
                                tunnel: w3235 -> [w3236]
                                frame #0 {
                                n2124 = property on="Trap Pos FB SP" class="DigNum (strict)"("Val(Sgnl)"=w3236) -> ()  [unwired: 2 in, 2 out]
                                }
                                frame #1 {
                                n2125 = Wait (ms)(milliseconds to wait=u32 700) -> ()  [unwired: 1 out]
                                }
                                frame #2 {
                                n2126 = local read "Action (%)"() -> (w3241:dbl)
                                n2127 = Absolute Value(x=w3241) -> (abs(x)=w3240:dbl)
                                n2128 = Greater?(x=w3240, y=70.0) -> (0:w3238:bool)
                                n2129 = property on="Remove Action Offset" class="Bool (strict)"("Val(Sgnl)"=w3238) -> ()  [unwired: 2 in, 2 out]
                                }
                                frame #3 {
                                n2130 = for {
                                N: 4 -> [_]
                                n2131 = flat-sequence {
                                frame #0 {
                                n2132 = Wait (ms)(milliseconds to wait=u32 500) -> ()  [unwired: 1 out]
                                }
                                frame #1 {
                                n2133 = local read "Action (%)"() -> (w3247:dbl)
                                n2134 = Absolute Value(x=w3247) -> (abs(x)=w3246:dbl)